vi "青蛙歷險記.vi"() -> ()   [LabVIEW 2014]
panel:
  in  "OK Button 2":bool
  in  "OK Button":bool
  out "Color Box 4":u32(colorbox)
  out "Color Box 7":u32(colorbox)
  out "sun":bool
  out "Color Box 5":u32(colorbox)
  out "Color Box 3":u32(colorbox)
  out "Color Box":u32(colorbox)
  out "result":bool
  out "5 X":bool
  out "4 X":bool
  out "3 X":bool
  out "2 X":bool
  out "1 X":bool
  out "Array 2":bool[](array[boolean])
  out "LAva":bool
  out "LAVA":bool
  out "x .and. y?":bool
  out "superman":bool
  out "Array name":string[](array[string])
  out "死幾次":i32[](array[numeric])
  out "幾P":i32
  out "DEAD":bool
  in  "SAVE ZONE":bool
  in  "JUMP":bool
  out "frog":bool
  in  "Slide":dbl(slide) scale=1.0..100.0
  out "Color Box 2":u32(colorbox)
  out "Color Box 6":u32(colorbox)
  out "Color Box 8":u32(colorbox)
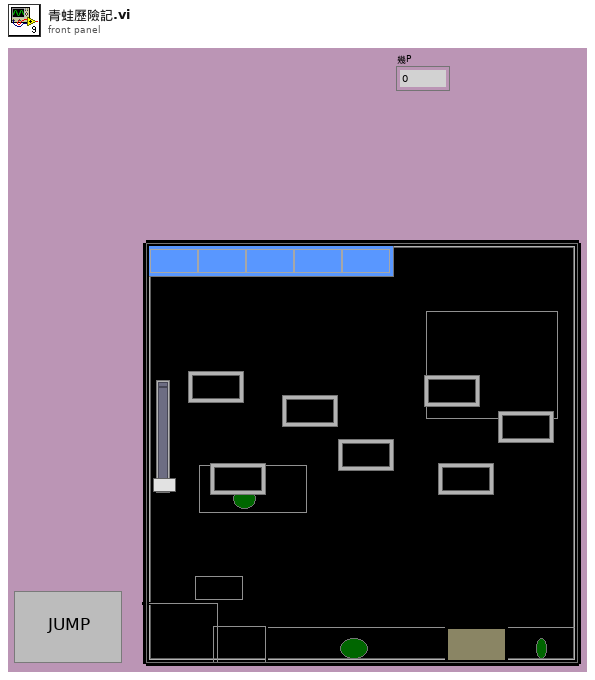
[diagram p1: front panel]
types:
  T1 = enum16{"init", "game", "easy", "hard", "result", "end", ""}
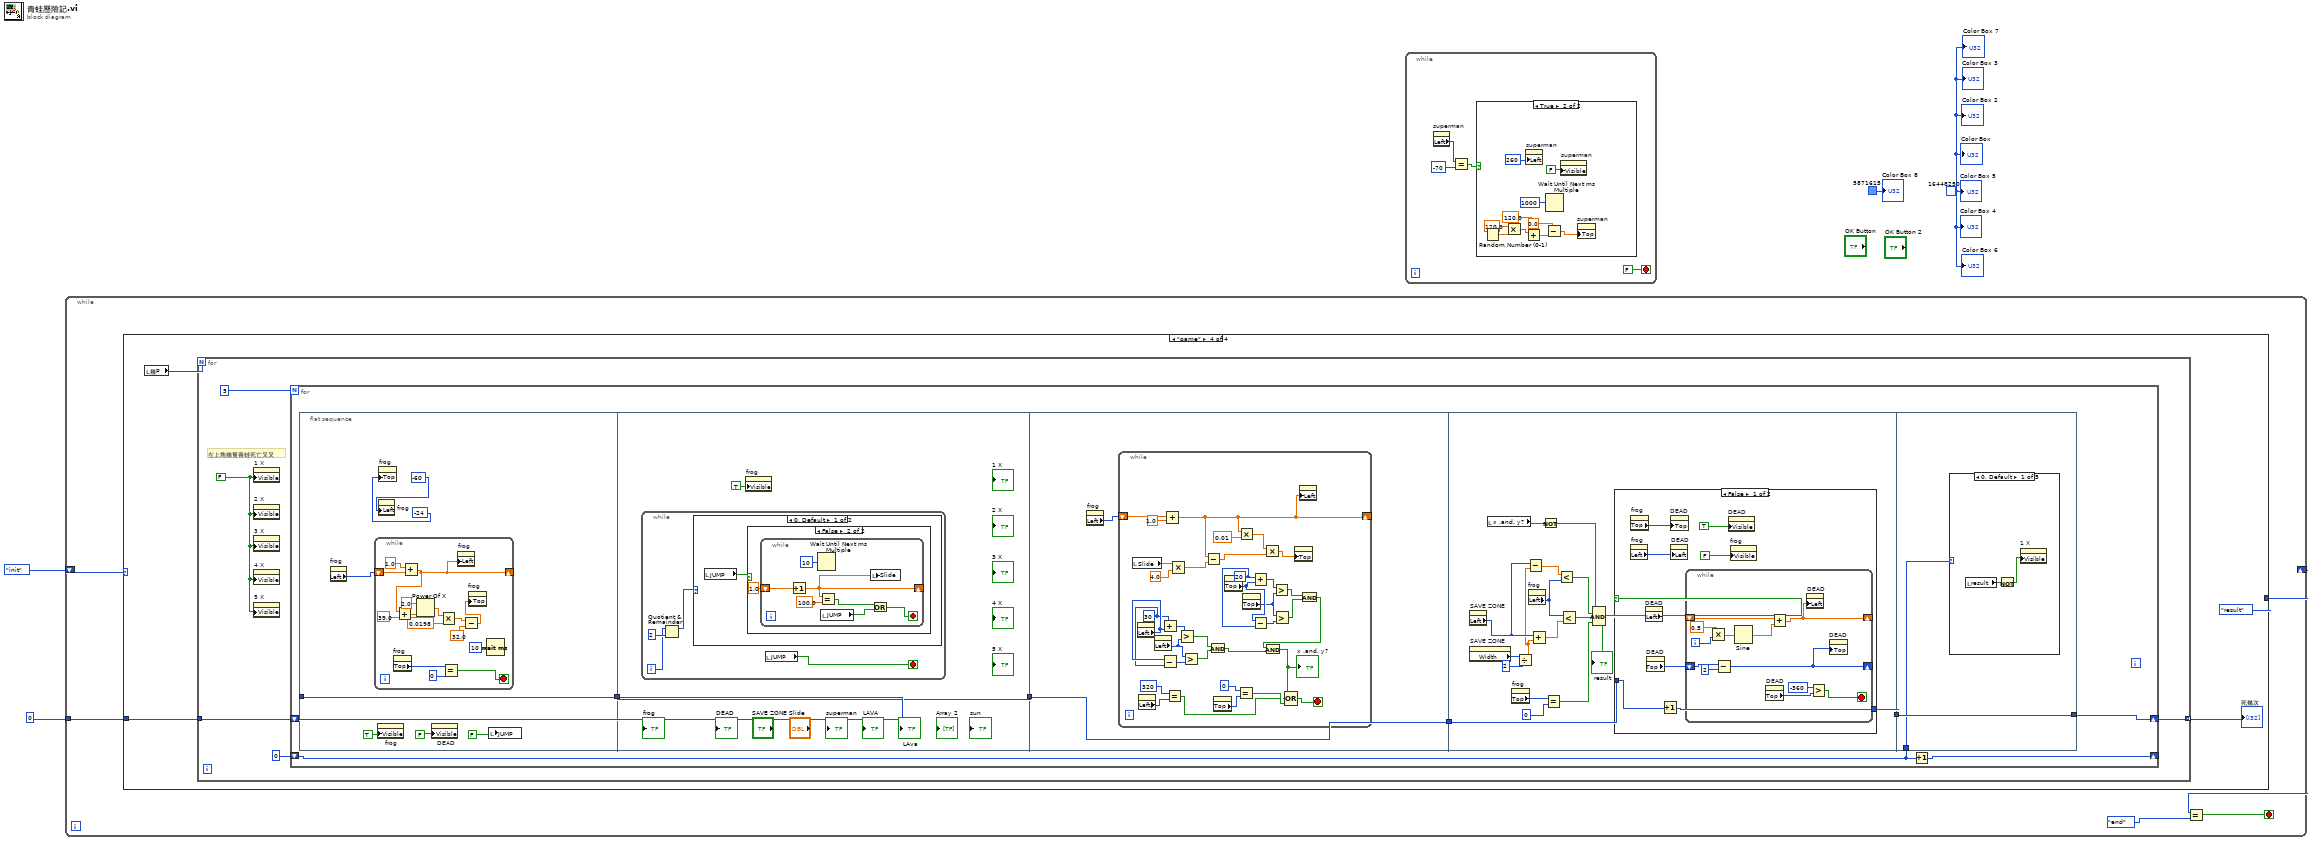
[diagram p0: block diagram]
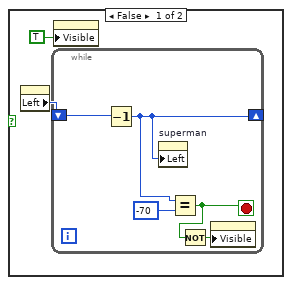
[diagram p2: hidden frame]
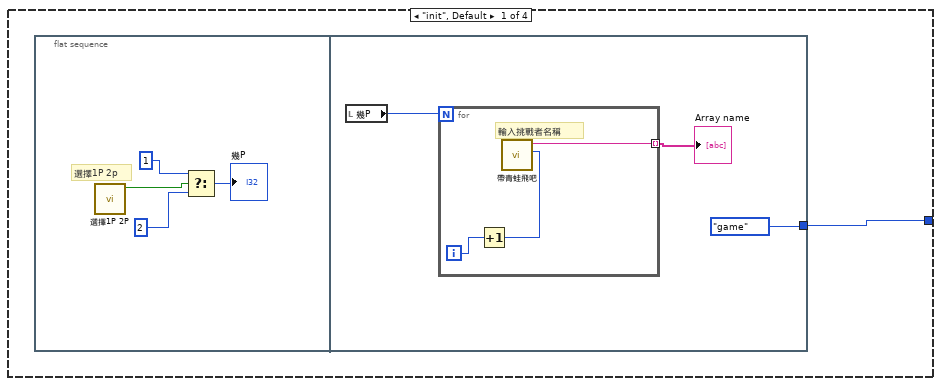
[diagram p3: hidden frame]
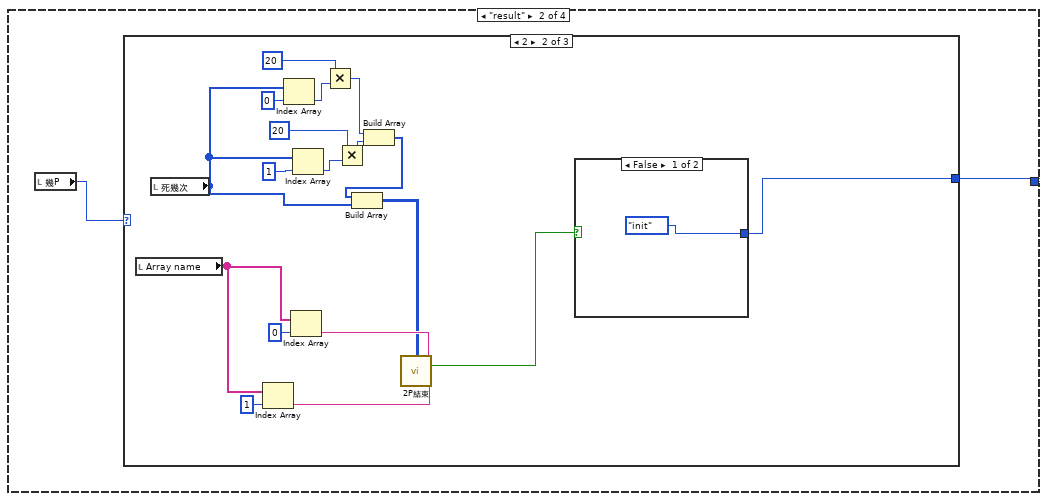
[diagram p4: hidden frame]
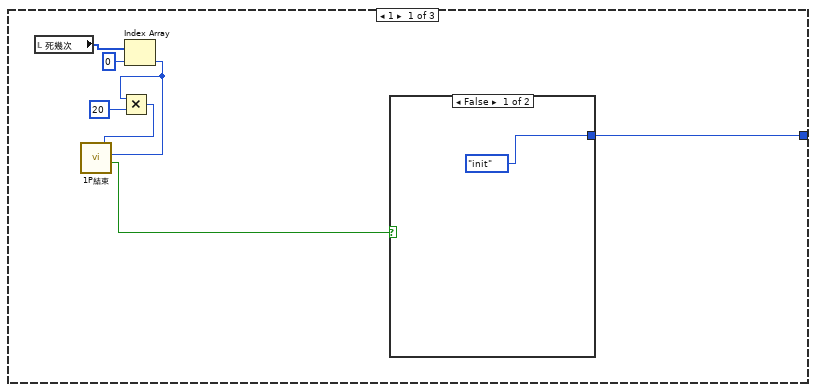
[diagram p5: hidden frame]
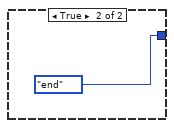
[diagram p6: hidden frame]
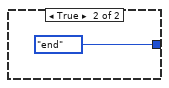
[diagram p7: hidden frame]
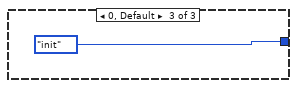
[diagram p8: hidden frame]
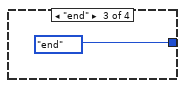
[diagram p9: hidden frame]
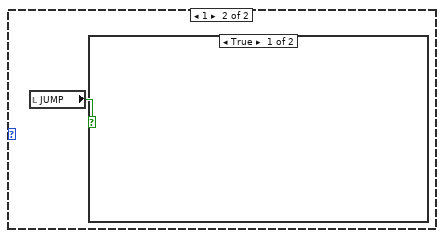
[diagram p11: hidden frame]
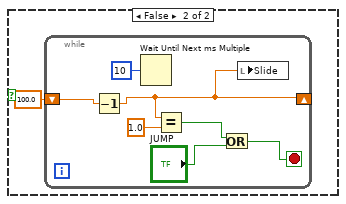
[diagram p12: hidden frame]
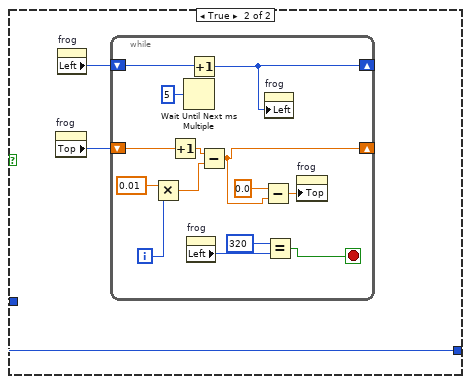
[diagram p13: hidden frame]
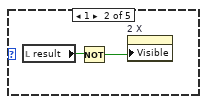
[diagram p14: hidden frame]
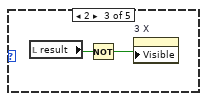
[diagram p15: hidden frame]
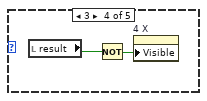
[diagram p16: hidden frame]
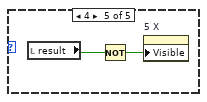
[diagram p17: hidden frame]
diagram:
  w1 = u32 16448250 ("Color Box 5")
  n1 = while {
    tunnel: 0 -> [w8]
    shift-right: [w6] -> _
    shift-left: T1."init" -> [w9]
    stop <- w5 stop-if-true
    n2 = case shown="\"game\"" w9 {
      tunnel: w8 -> [_ _ _ w55]
      tunnel: [w10 w21 T1."end" T1."result"] -> w6
      frame "init", Default {
        n3 = flat-sequence {
          tunnel: [T1."game"] -> w10
          frame #0 {
            # "選擇1P 2p"
            n4 = call "選擇1P 2P.vi"() -> ("OK Button 3"=w14:bool)  [unwired: 10 in, 1 out]
            n5 = Select(t=1, s=w14, f=2) -> (s? t:f=→"幾P":i32)
          }
          frame #1 {
            n6 = local read "幾P"() -> (w17:i32)
            n7 = for {
              N: w17 -> [_]
              tunnel: [w20] -> w16 mode=indexing
              i -> [w19]
              # "輸入挑戰者名稱"
              n8 = Increment(x=w19) -> (x+1=w18:i32)
              n9 = call "帶青蛙飛吧.vi"("Numeric"=w18) -> ("英勇的挑戰者請輸入名稱: 2"=w20:string)  [unwired: 10 in]
            }
            "Array name" <- w16
          }
        }
      }
      frame "result" {
        n10 = local read "幾P"() -> (w22:i32)
        n11 = case shown="2" w22 {
          tunnel: [w29 w36 T1."init"] -> w21
          frame 1 {
            n12 = local read "死幾次"() -> (w28:i32[])
            n13 = Index Array(array=w28, index=0) -> (element=w26:i32)
            n14 = Multiply(x=w26, y=20) -> (x*y=w24:i32)
            n15 = call "1P結束.vi"("青蛙數"=w26, "您的分數"=w24) -> ("結束 2"=w23:bool)  [unwired: 7 in]
            n16 = case shown="False" w23 {
              tunnel: [T1."init" T1."end"] -> w29
              frame False {
              }
              frame True {
              }
            }
          }
          frame 2 {
            n17 = local read "Array name"() -> (w48:string[])
            n18 = local read "死幾次"() -> (w45:i32[])
            n19 = Index Array(array=w48, index=1) -> (element=w34:string)
            n20 = Index Array(array=w45, index=0) -> (element=w42:i32)
            n21 = Index Array(array=w48, index=0) -> (element=w35:string)
            n22 = Index Array(array=w45, index=1) -> (element=w39:i32)
            n23 = Multiply(x=20, y=w42) -> (x*y=w40:i32)
            n24 = Multiply(x=20, y=w39) -> (x*y=w37:i32)
            n25 = Build Array(w40, w37) -> (w43:i32[])
            n26 = Build Array(w43, w45) -> (w33:i32[][])
            n27 = call "2P結束.vi"("Array"=w33, "String 2"=w34, "String"=w35) -> ("final 2"=w32:bool)  [unwired: 7 in, 1 out]
            n28 = case shown="False" w32 {
              tunnel: [T1."init" T1."end"] -> w36
              frame False {
              }
              frame True {
              }
            }
          }
          frame 0, Default {
          }
        }
      }
      frame "end" {
      }
      frame "game" {
        n29 = local read "幾P"() -> (w56:i32)
        n30 = for {
          N: w56 -> [_]
          tunnel: w55 -> [w61]
          tunnel: [w60] -> w57 mode=indexing
          w59 = FALSE ("Visible")
          # "左上角幾隻青蛙死亡叉叉"
          n31 = property on="1 X" class="Bool (strict)"("Visible"=w59) -> ()  [unwired: 2 in, 2 out]
          n32 = property on="2 X" class="Bool (strict)"("Visible"=w59) -> ()  [unwired: 2 in, 2 out]
          n33 = property on="3 X" class="Bool (strict)"("Visible"=w59) -> ()  [unwired: 2 in, 2 out]
          n34 = property on="4 X" class="Bool (strict)"("Visible"=w59) -> ()  [unwired: 2 in, 2 out]
          n35 = property on="5 X" class="Bool (strict)"("Visible"=w59) -> ()  [unwired: 2 in, 2 out]
          n36 = for {
            N: 5 -> [_]
            shift-right: [w66] -> w60
            shift-left: w61 -> [w70]
            shift-right: [w64] -> _
            shift-left: 0 -> [w63]
            n37 = flat-sequence {
              tunnel: w70 -> [w74]
              tunnel: [w74] -> w67
              tunnel: [w93] -> w68
              tunnel: w67 -> [w93]
              tunnel: [w117] -> w69
              tunnel: w68 -> [w117]
              tunnel: w69 -> [w156]
              tunnel: [w155] -> w65
              tunnel: [w208] -> w66
              tunnel: w65 -> [w208]
              tunnel: w63 -> [w207]
              frame #0 {
                n38 = property on="frog" class="Bool (strict)"() -> ("Left"=w71:i32)  [unwired: 2 in, 2 out]
                n39 = while {
                  shift-right: [w80] -> _
                  shift-left: w71 -> [w92]
                  stop <- w82 stop-if-true
                  n40 = property on="frog" class="Bool (strict)"() -> ("Top"=w78:i32)  [unwired: 2 in, 2 out]
                  n41 = Add(x=1.0, y=w92) -> (x+y=w80:dbl)
                  n42 = Add(x=w80, y=39.0) -> (x+y=w89:dbl)
                  n43 = Power Of X(1:w89, 2:2.0 ("y")) -> (0:w87:dbl)
                  n44 = Multiply(x=w87, y=0.0198) -> (x*y=w85:dbl)
                  n45 = Equal?(x=w78, y=0) -> (x = y?=w82:bool)
                  n46 = property on="frog" class="Bool (strict)"("Left"=w80) -> ()  [unwired: 2 in, 2 out]
                  n47 = Subtract(x=w85, y=32.0) -> (x-y=w79:dbl)
                  n48 = property on="frog" class="Bool (strict)"("Top"=w79) -> ()  [unwired: 2 in, 2 out]
                  n49 = Wait (ms)(milliseconds to wait=u32 10) -> ()  [unwired: 1 out]
                }
                n50 = property on="frog" class="Bool (strict)"("Visible"=TRUE) -> ()  [unwired: 2 in, 2 out]
                n51 = property on="frog" class="Bool (strict)"("Left"=-60 ("Position:Left")) -> ()  [unwired: 2 in, 2 out]
                n52 = property on="frog" class="Bool (strict)"("Top"=-24 ("Position:Top")) -> ()  [unwired: 2 in, 2 out]
                n53 = property on="DEAD" class="Bool (strict)"("Visible"=FALSE) -> ()  [unwired: 2 in, 2 out]
                n54 = local write "JUMP"(FALSE ("OK Button")) -> ()
              }
              frame #1 {
                n55 = while {
                  i -> [w97]
                  stop <- w95 stop-if-true
                  n56 = Quotient & Remainder(x=w97, y=2) -> (x-y*floor(x/y)=w96:i32)  [unwired: 1 out]
                  n57 = case shown="0, Default" w96 {
                    frame 0, Default {
                      n58 = local read "JUMP"() -> (w99:bool)
                      n59 = case shown="False" w99 {
                        frame True {
                        }
                        frame False {
                          n60 = while {
                            shift-right: [w106] -> _
                            shift-left: 1.0 -> [w107]
                            stop <- w101 stop-if-true
                            n61 = Increment(x=w107) -> (x+1=w106:dbl)
                            n62 = Wait Until Next ms Multiple(millisecond multiple=u32 10) -> ()  [unwired: 1 out]
                            n63 = Equal?(x=w106, y=100.0) -> (x = y?=w102:bool)
                            n64 = local read "JUMP"() -> (w103:bool)
                            n65 = local write "Slide"(w106) -> ()
                            n66 = Or(x=w102, y=w103) -> (x .or. y?=w101:bool)
                          }
                        }
                      }
                    }
                    frame 1 {
                      n67 = local read "JUMP"() -> (w108:bool)
                      n68 = case shown="True" w108 {
                        frame True {
                        }
                        frame False {
                          n69 = while {
                            shift-right: [w110] -> _
                            shift-left: 100.0 -> [w111]
                            stop <- w113 stop-if-true
                            n70 = Decrement(x=w111) -> (x-1=w110:dbl)
                            n71 = Wait Until Next ms Multiple(millisecond multiple=u32 10) -> ()  [unwired: 1 out]
                            n72 = Equal?(x=w110, y=1.0) -> (x = y?=w114:bool)
                            n73 = Or(x=w114, y="JUMP") -> (x .or. y?=w113:bool)
                            n74 = local write "Slide"(w110) -> ()
                          }
                        }
                      }
                    }
                  }
                  n75 = local read "JUMP"() -> (w95:bool)
                }
                n76 = property on="frog" class="Bool (strict)"("Visible"=TRUE) -> ()  [unwired: 2 in, 2 out]
              }
              frame #2 {
                n77 = property on="frog" class="Bool (strict)"() -> ("Left"=w118:i32)  [unwired: 2 in, 2 out]
                n78 = while {
                  shift-right: [w143] -> _
                  shift-left: w118 -> [w151]
                  stop <- w120 stop-if-true
                  w131 = 20 ("x")
                  w136 = 30 ("x")
                  n79 = local read "Slide"() -> (w146:dbl)
                  n80 = property on="superman" class="Bool (strict)"() -> ("Left"=w138:i32)  [unwired: 2 in, 2 out]
                  n81 = property on="frog" class="Bool (strict)"() -> ("Left"=w148:i32)  [unwired: 2 in, 2 out]
                  n82 = property on="frog" class="Bool (strict)"() -> ("Left"=w135:i32)  [unwired: 2 in, 2 out]
                  n83 = Add(x=w136, y=w138) -> (x+y=w137:i32)
                  n84 = Subtract(x=w138, y=w136) -> (x-y=w134:i32)
                  n85 = Add(x=w151, y=1.0) -> (x+y=w143:dbl)
                  n86 = Equal?(x=320, y=w148) -> (x = y?=w124:bool)
                  n87 = Multiply(x=w146, y=4.0) -> (x*y=w144:dbl)
                  n88 = Greater?(x=w137, y=w135) -> (0:w133:bool)
                  n89 = Greater?(x=w135, y=w134) -> (0:w132:bool)
                  n90 = Subtract(x=w143, y=w144) -> (x-y=w140:dbl)
                  n91 = And(x=w133, y=w132) -> (x .and. y?=w123:bool)
                  n92 = property on="frog" class="Bool (strict)"() -> ("Top"=w149:i32)  [unwired: 2 in, 2 out]
                  n93 = property on="superman" class="Bool (strict)"() -> ("Top"=w129:i32)  [unwired: 2 in, 2 out]
                  n94 = Equal?(x=0, y=w149) -> (x = y?=w125:bool)
                  n95 = Multiply(x=w143, y=0.01) -> (x*y=w141:dbl)
                  n96 = property on="frog" class="Bool (strict)"() -> ("Top"=w128:i32)  [unwired: 2 in, 2 out]
                  n97 = Add(x=w131, y=w129) -> (x+y=w130:i32)
                  n98 = Subtract(x=w129, y=w131) -> (x-y=w119:i32)
                  n99 = Multiply(x=w141, y=w140) -> (x*y=w139:dbl)
                  n100 = Greater?(x=w130, y=w128) -> (0:w127:bool)
                  n101 = Greater?(x=w128, y=w119) -> (0:w126:bool)
                  n102 = property on="frog" class="Bool (strict)"("Top"=w139) -> ()  [unwired: 2 in, 2 out]
                  n103 = property on="frog" class="Bool (strict)"("Left"=w143) -> ()  [unwired: 2 in, 2 out]
                  n104 = And(x=w127, y=w126) -> (x .and. y?=w122:bool)
                  n105 = And(x=w122, y=w123) -> (x .and. y?=w121:bool)
                  "x .and. y?" <- w121
                  n106 = Compound Arithmetic op=OR(w121, w124, w125) -> (w120:bool)
                }
              }
              frame #3 {
                n107 = property on="SAVE ZONE" class="Bool"() -> ("Left"=w166:i32)  [unwired: 2 in, 2 out]
                n108 = property on="SAVE ZONE" class="Bool"() -> ("Width"=w169:u32)  [unwired: 2 in, 2 out]
                n109 = local read "x .and. y?"() -> (w154:bool)
                n110 = property on="frog" class="Bool (strict)"() -> ("Top"=w162:i32)  [unwired: 2 in, 2 out]
                n111 = Divide(x=w169, y=u32 2) -> (x/y=w165:dbl)
                n112 = Subtract(x=w166, y=w165) -> (x-y=w164:dbl)
                n113 = property on="frog" class="Bool (strict)"() -> ("Left"=w163:i32)  [unwired: 2 in, 2 out]
                n114 = Add(x=w166, y=w165) -> (x+y=w167:dbl)
                n115 = Not(x=w154) -> (.not. x?=w153:bool)
                n116 = Equal?(x=w162, y=0) -> (x = y?=w158:bool)
                n117 = Less?(x=w164, y=w163) -> (x < y?=w160:bool)
                n118 = Less?(x=w163, y=w167) -> (x < y?=w159:bool)
                n119 = Compound Arithmetic op=AND(w153, w160, w159, w158) -> (w157:bool)
                "result" <- w157
                n120 = case shown="False" w157 {
                  tunnel: w156 -> [w171 w190]
                  tunnel: [w170 w190] -> w155
                  frame False {
                    n121 = property on="frog" class="Bool (strict)"() -> ("Top"=w177:i32)  [unwired: 2 in, 2 out]
                    n122 = property on="frog" class="Bool (strict)"() -> ("Left"=w176:i32)  [unwired: 2 in, 2 out]
                    n123 = property on="DEAD" class="Bool (strict)"() -> ("Left"=w174:i32)  [unwired: 2 in, 2 out]
                    n124 = property on="DEAD" class="Bool (strict)"() -> ("Top"=w173:i32)  [unwired: 2 in, 2 out]
                    n125 = Increment(x=w171) -> (x+1=w170:i32)
                    n126 = property on="DEAD" class="Bool (strict)"("Top"=w177) -> ()  [unwired: 2 in, 2 out]
                    n127 = property on="DEAD" class="Bool (strict)"("Left"=w176) -> ()  [unwired: 2 in, 2 out]
                    n128 = while {
                      shift-right: [w182] -> _
                      shift-left: w174 -> [w189]
                      shift-right: [w180] -> _
                      shift-left: w173 -> [w179]
                      i -> [w187]
                      stop <- w183 stop-if-true
                      n129 = Multiply(x=0.5, y=w187) -> (x*y=w185:dbl)
                      n130 = Subtract(x=w179, y=2) -> (x-y=w180:i32)
                      n131 = Sine(x=w185) -> (sin(x)=w188:dbl)
                      n132 = property on="DEAD" class="Bool (strict)"() -> ("Top"=w181:i32)  [unwired: 2 in, 2 out]
                      n133 = Add(x=w189, y=w188) -> (x+y=w182:dbl)
                      n134 = property on="DEAD" class="Bool (strict)"("Left"=w182) -> ()  [unwired: 2 in, 2 out]
                      n135 = Greater?(x=-360, y=w181) -> (0:w183:bool)
                      n136 = property on="DEAD" class="Bool (strict)"("Top"=w180) -> ()  [unwired: 2 in, 2 out]
                    }
                    n137 = property on="DEAD" class="Bool (strict)"("Visible"=TRUE) -> ()  [unwired: 2 in, 2 out]
                    n138 = property on="frog" class="Bool (strict)"("Visible"=FALSE) -> ()  [unwired: 2 in, 2 out]
                  }
                  frame True {
                    n139 = property on="frog" class="Bool (strict)"() -> ("Top"=w191:i32)  [unwired: 2 in, 2 out]
                    n140 = property on="frog" class="Bool (strict)"() -> ("Left"=w192:i32)  [unwired: 2 in, 2 out]
                    n141 = while {
                      shift-right: [w202] -> _
                      shift-left: w192 -> [w206]
                      shift-right: [w194] -> _
                      shift-left: w191 -> [w201]
                      i -> [w199]
                      stop <- w203 stop-if-true
                      n142 = Multiply(x=0.01, y=w199) -> (x*y=w197:dbl)
                      n143 = Increment(x=w201) -> (x+1=w200:dbl)
                      n144 = Wait Until Next ms Multiple(millisecond multiple=u32 5) -> ()  [unwired: 1 out]
                      n145 = property on="frog" class="Bool (strict)"() -> ("Left"=w205:i32)  [unwired: 2 in, 2 out]
                      n146 = Increment(x=w206) -> (x+1=w202:i32)
                      n147 = Subtract(x=w200, y=w197) -> (x-y=w194:dbl)
                      n148 = Subtract(x=0.0, y=w194) -> (x-y=w196:dbl)
                      n149 = property on="frog" class="Bool (strict)"("Left"=w202) -> ()  [unwired: 2 in, 2 out]
                      n150 = Equal?(x=320, y=w205) -> (x = y?=w203:bool)
                      n151 = property on="frog" class="Bool (strict)"("Top"=w196) -> ()  [unwired: 2 in, 2 out]
                    }
                  }
                }
              }
              frame #4 {
                n152 = case shown="0, Default" w207 {
                  frame 0, Default {
                    n153 = local read "result"() -> (w209:bool)
                    n154 = Not(x=w209) -> (.not. x?=w210:bool)
                    n155 = property on="1 X" class="Bool (strict)"("Visible"=w210) -> ()  [unwired: 2 in, 2 out]
                  }
                  frame 1 {
                    n156 = local read "result"() -> (w212:bool)
                    n157 = Not(x=w212) -> (.not. x?=w211:bool)
                    n158 = property on="2 X" class="Bool (strict)"("Visible"=w211) -> ()  [unwired: 2 in, 2 out]
                  }
                  frame 2 {
                    n159 = local read "result"() -> (w213:bool)
                    n160 = Not(x=w213) -> (.not. x?=w214:bool)
                    n161 = property on="3 X" class="Bool (strict)"("Visible"=w214) -> ()  [unwired: 2 in, 2 out]
                  }
                  frame 3 {
                    n162 = local read "result"() -> (w215:bool)
                    n163 = Not(x=w215) -> (.not. x?=w216:bool)
                    n164 = property on="4 X" class="Bool (strict)"("Visible"=w216) -> ()  [unwired: 2 in, 2 out]
                  }
                  frame 4 {
                    n165 = local read "result"() -> (w217:bool)
                    n166 = Not(x=w217) -> (.not. x?=w218:bool)
                    n167 = property on="5 X" class="Bool (strict)"("Visible"=w218) -> ()  [unwired: 2 in, 2 out]
                  }
                }
              }
            }
            n168 = Increment(x=w63) -> (x+1=w64:i32)
          }
        }
        "死幾次" <- w57
      }
    }
    n169 = Equal?(x=w6, y=T1."end") -> (x = y?=w5:bool)
  }
  n170 = while {
    stop <- FALSE stop-if-true
    n171 = property on="superman" class="Bool (strict)"() -> ("Left"=w222:i32)  [unwired: 2 in, 2 out]
    n172 = Equal?(x=w222, y=-70) -> (x = y?=w220:bool)
    n173 = case shown="True" w220 {
      frame False {
        n174 = property on="superman" class="Bool (strict)"() -> ("Left"=w224:i32)  [unwired: 2 in, 2 out]
        n175 = while {
          shift-right: [w228] -> _
          shift-left: w224 -> [w229]
          stop <- w226 stop-if-true
          n176 = Decrement(x=w229) -> (x-1=w228:i32)
          n177 = property on="superman" class="Bool (strict)"("Left"=w228) -> ()  [unwired: 2 in, 2 out]
          n178 = Equal?(x=w228, y=-70) -> (x = y?=w226:bool)
          n179 = Not(x=w226) -> (.not. x?=w225:bool)
          n180 = property on="superman" class="Bool (strict)"("Visible"=w225) -> ()  [unwired: 2 in, 2 out]
        }
        n181 = property on="superman" class="Bool (strict)"("Visible"=TRUE) -> ()  [unwired: 2 in, 2 out]
      }
      frame True {
        n182 = Random Number (0-1)() -> (number: 0 to 1=w231:dbl)
        n183 = Multiply(x=120.0, y=w231) -> (x*y=w233:dbl)
        n184 = Add(x=w233, y=120.0) -> (x+y=w235:dbl)
        n185 = property on="superman" class="Bool (strict)"("Left"=260 ("Position:Left")) -> ()  [unwired: 2 in, 2 out]
        n186 = Wait Until Next ms Multiple(millisecond multiple=u32 1000) -> ()  [unwired: 1 out]
        n187 = Subtract(x=0.0, y=w235) -> (x-y=w230:dbl)
        n188 = property on="superman" class="Bool (strict)"("Visible"=FALSE) -> ()  [unwired: 2 in, 2 out]
        n189 = property on="superman" class="Bool (strict)"("Top"=w230) -> ()  [unwired: 2 in, 2 out]
      }
    }
  }
  "Color Box" <- w1
  "Color Box 2" <- w1
  "Color Box 3" <- w1
  "Color Box 4" <- w1
  "Color Box 5" <- w1
  "Color Box 6" <- w1
  "Color Box 8" <- u32 5871615 ("Color Box 8")
  "Color Box 7" <- w1
